vi "UHR-Fleezers Control (host) - 12.7e.vi"() -> ()   [LabVIEW 2012] (continued)
  T23 = typedef "XDNodeRunTimeDep.lvlib/timing_clust.ctl" = cluster{"Expected End [f-1]":u64, "Actual End [f-1]":u64, "Finished Late? [f-1]":bool, "Expected End [i-1]":u64, "Actual End [i-1]":u64, "Finished Late? [i-1]":bool, "Expected Start [i]":u64, "Actual Start [i]":u64, "Expected Start [f]":u64, "Actual Start [f]":u64, "Source Name":string, "Structure Name":string, "Period":i64, "Deadline":i64, "Offset":i64, "Start":i64, "Priority":i32, "Timeout":i32, "Mode":T24, "Wakeup Reason":T25, "Error":errorcluster, "Source Type":string, "Secondary Source Type":string, "Global End Time":u64, "Global Start Time":u64, "Frame Duration":u64, "Iteration Duration":u64, "Assigned CPU":i32, "I/O Scan Engine Mode":u32}
  T24 = typedef "XDNodeRunTimeDep.lvlib/nitl_modes.ctl" = enum32{"No Change", "Process missed periods, maintain original phase", "Discard missed periods, maintain original phase", "Process missed periods, ignore original phase", "Discard missed periods, ignore original phase"}
  T25 = typedef "XDNodeRunTimeDep.lvlib/wakeup.ctl" = enum32{"Normal", "Aborted", "Asynchronous wakeup", "Timing source error", "Timed loop error", "Timeout"}
  T26 = enum16{"big-endian, network order", "native, host order", "little-endian"}
  T27 = enum16{"open", "replace", "create", "open or create", "replace or create", "replace or create with confirmation"}
  T28 = cluster{"Scan Range AOD (nm) 2":dbl, "Step Size AOD (nm) 2":dbl, "Scan Speed AOD (nm/s) 2":dbl, "Number of scans (AOD) 2":u16, "Label":string}
  T29 = cluster{"[0]":dbl, "[1]":dbl, "[2]":dbl, "[3]":dbl, "[4]":dbl, "[5]":dbl}
  T30 = cluster{"Diameter (mm)":dbl, "Units":dbl, "Volume":dbl, "Rate":dbl}
  T31 = enum32{"Status", "Sample Stage", "Syringe Pump", "Trap Control (RF)", "APD Counting", "Fluorescence Laser Control", "Trap AI", "Video", "FPGA"}
  T32 = enum32{"Status", "Sample Stage", "Syringe Pump", "Trap Control (RF)", "APD Counting", "Fluorescence Laser Control", "Trap AI", "Video", "FPGA", "Misc. Configuration"}
  T33 = cluster{"Left":i32, "Top":i32, "Width":u32, "Height":u32}
  T34 = cluster{cluster{"Left":i32, "Top":i32, "Width":u32, "Height":u32}}[]
  T35 = enum32{"setting", "request", "request control", "info", "statistics", "system settings", "I/O sub system", "HRT control", "camera descriptions", "device specific data", "event sub system settings", "event sub system results", "image memory manager"}
  T36 = typedef "AviRefnum.ctl" = refnum<k1>
  T37 = typedef "imagedata.ctl" = cluster{"image type":i32, "image depth":i32, "image":u8[], "mask":u8[], "colors":u32[], "Rectangle":cluster{"left":i16, "top":i16, "right":i16, "bottom":i16}}
  T38 = enum32{"Normal Display", "Dual Display (APD)", "FFT", "High Res Display"}
  T39 = cluster{"Origin Pixel":cluster{"X":sgl, "Y":sgl}, "Angle Relative to Horizontal (deg)":sgl, "Axis Reference":u32}
  T40 = typedef "Simple Grid Descriptor" = cluster{"X Step":sgl, "Y Step":sgl, "Unit":T41}
  T41 = typedef "Image Unit" = enum32{"Undefined", "Angström", "Micrometer", "Millimeter", "Centimeter", "Meter", "Kilometer", "Microinch", "Inch", "Feet", "Nautical miles", "Standard miles", "Steps"}
  T42 = cluster{"averaging mode":u16, "weighting mode":u16, "number of averages":u32}
  T43 = cluster{"dB On (F)":bool, "unwrap phase (F)":bool, "convert to degree (F)":bool}
  T44 = cluster{string, string, string, string, string, string, string, string}
  T45 = cluster{string, string, string, string, string, string, string, string, string, string, string, string}
  T46 = cluster{string, string, string, string, string, string, string, string, string, string, string, string, string}
  T47 = cluster{string, string, string, string, string, string, string, string, string, string, string, string, string, string}
  T48 = cluster{"BD 1 Frequency 1 (MHz)":dbl, "BD 1 Frequency 2 (MHz)":dbl}
  T49 = cluster{"f0":dbl, "df":dbl, "magnitude":dbl[]}[][]
  T50 = cluster{"Comment (data description)":string, "Channel 1 Buffer":string, "Channel 2 Buffer":string, "Channel 3 Buffer":string, "Title":string, "DNA Construct":string, "Bead diameter":dbl, "Name":string}
diagram:
  w18 = u16 10 items=["1.0"=10, "1.5"=15, "2.0"=20] ("stop bits (10: 1 bit)")
  w34 = u16 20 items=["1.0"=10, "1.5"=15, "2.0"=20] ("stop bits (10: 1 bit)")
  w37 = u16 20 items=["1.0"=10, "1.5"=15, "2.0"=20] ("stop bits (10: 1 bit)")
  w45 = u16 20 items=["1.0"=10, "1.5"=15, "2.0"=20] ("stop bits (10: 1 bit)")
  w24 = T19 2 items=["Grayscale (U8)", "Grayscale (I16)", "Grayscale (SGL)", "Complex (CSG)", "RGB (U32)", "HSL (U32)", "RGB (U64)", "Grayscale (U16)"] ("Image Type")
  # "Settings to help prevent AOM/D damage"
  # "Initialize the FPGA DAQ card itself"
  # "Reset the DAQ card."
  # "Specify the DAQ card and the FPGA code to run"
  # "Bottom 1 Harvard"
  # "Top 3 Harvard"
  # "Center Harvard"
  # "Bottom 1 Harvard"
  # "Top 3 Harvard"
  # "Center Harvard"
  n1 = case "Trap X limits" shown="\"AOD3Sets\"" "1axis AOM vs 2 axis AOD" {
    tunnel: [T16 {"Minimum"=0.0, "Maximum"=40.0, "Increment"=0.1} ("Min Max Inc") T16 {"Minimum"=0.0, "Maximum"=40.0, "Increment"=0.1} ("Min Max Inc") T16 {"Minimum"=60.0, "Maximum"=90.0, "Increment"=1.0} ("Min Max Inc")] -> w9
    tunnel: [T16 {"Minimum"=0.0, "Maximum"=45.0, "Increment"=1.0} ("Data Entry Limits") T16 {"Minimum"=0.0, "Maximum"=45.0, "Increment"=1.0} ("Data Entry Limits") T16 {"Minimum"=0.0, "Maximum"=50.0, "Increment"=1.0} ("Data Entry Limits")] -> w7
    frame "2axisAOD" {
      w81 = u16 300 ("DIO count 1 (ticks)")
      # "Amp Limits"
      # "Freq Limits"
      n2 = disable-structure shown="Disabled" {
        frame Disabled {
          w87 = 35.0 ("BD 1 Amplitude 1 (%)")
          w88 = 30.0 ("BD 1 Frequency 1 (MHz)")
          n3 = local write "BD 1 Frequency 1 (MHz)"(w88) -> ()
          n4 = local write "BD 1 Frequency 2 (MHz)"(w88) -> ()
          n5 = local write "BD 1 Amplitude 2 (%)"(w87) -> ()
          n6 = local write "BD 1 Amplitude 1 (%)"(w87) -> ()
          n7 = local write "BD 2 Frequency 1 (MHz)"(w88) -> ()
          n8 = local write "BD 2 Amplitude 1 (%)"(w87) -> ()
          n9 = local write "BD 2 Frequency 2 (MHz)"(w88) -> ()
          n10 = local write "BD 2 Amplitude 2 (%)"(w87) -> ()
        }
        frame Enabled {
        }
      }
      n11 = local write "All FB On/Off"(FALSE ("All FB On/Off")) -> ()
      n12 = local write "BD 2 Delay (Ticks)"(u8 108 ("BD 2 Delay (Ticks)")) -> ()
      n13 = local write "Number Interlace Sets"(u8 2 ("Number Interlace Sets")) -> ()
      n14 = local write "DIO count 2 (ticks)"(w81) -> ()
      n15 = local write "DIO count 1 (ticks)"(w81) -> ()
    }
    frame "AOD3Sets" {
      w89 = u16 200 ("DIO count 1 (ticks)")
      # "Amp Limits"
      # "Freq Limits"
      n16 = disable-structure shown="Disabled" {
        frame Disabled {
          w95 = 35.0 ("BD 1 Amplitude 1 (%)")
          w96 = 30.0 ("BD 1 Frequency 1 (MHz)")
          n17 = local write "BD 1 Frequency 1 (MHz)"(w96) -> ()
          n18 = local write "BD 1 Frequency 2 (MHz)"(w96) -> ()
          n19 = local write "BD 1 Amplitude 2 (%)"(w95) -> ()
          n20 = local write "BD 1 Amplitude 1 (%)"(w95) -> ()
          n21 = local write "BD 2 Frequency 1 (MHz)"(w96) -> ()
          n22 = local write "BD 2 Amplitude 1 (%)"(w95) -> ()
          n23 = local write "BD 2 Frequency 2 (MHz)"(w96) -> ()
          n24 = local write "BD 2 Amplitude 2 (%)"(w95) -> ()
        }
        frame Enabled {
        }
      }
      n25 = local write "All FB On/Off"(FALSE ("All FB On/Off")) -> ()
      n26 = local write "BD 2 Delay (Ticks)"(u8 0 ("BD 2 Delay (Ticks)")) -> ()
      n27 = local write "Number Interlace Sets"(u8 3 ("Number Interlace Sets")) -> ()
      n28 = local write "DIO count 2 (ticks)"(w89) -> ()
      n29 = local write "DIO count 1 (ticks)"(w89) -> ()
    }
    frame "1axis", Default {
      # "Amp Lmits"
      # "Freq Limits"
    }
  }
  n30 = xnode "Open FPGA VI Reference"("resource name"=T18 "750kHzDAQ") -> ("FPGA VI Reference Out"=w14:T20, "error out"=w13:errorcluster)  [unwired: 1 in]
  n31 = xnode "Invoke Method"("FPGA VI Reference In"=w14, "error in"=w13) -> ("FPGA VI Reference Out"=w6:T20, "error out"=→"FPGA error out":errorcluster)
  n32 = flat-sequence "Safety limits on RF frequencies and amplitudes (for AOM protection)" {
    tunnel: [w101] -> w1
    tunnel: [w100] -> w3
    tunnel: [w102] -> w4
    tunnel: [w103] -> w2
    tunnel: w9 -> [w101]
    tunnel: w7 -> [w100]
    tunnel: w6 -> [w99]
    tunnel: [w99] -> w5
    frame #0 {
      w103 = T16 {"Minimum"=0.0, "Maximum"=40.0, "Increment"=0.1} ("Min Max Inc")
      w102 = T16 {"Minimum"=0.0, "Maximum"=45.0, "Increment"=1.0} ("Data Entry Limits")
      n33 = property on="BD 2 Frequency 1 (MHz)" class="DigNum (strict)"("Data Range"=w103) -> ()  [unwired: 2 in, 2 out]
      n34 = property on="BD 2 Frequency 3 (MHz)" class="DigNum (strict)"("Data Range"=w103) -> ()  [unwired: 2 in, 2 out]
      n35 = property on="BD 2 Frequency 2 (MHz)" class="DigNum (strict)"("Data Range"=w103) -> ()  [unwired: 2 in, 2 out]
      n36 = property on="BD 1 Frequency 1 (MHz)" class="DigNum (strict)"("Data Range"=w101) -> ()  [unwired: 2 in, 2 out]
      n37 = property on="BD 1 Frequency 2 (MHz)" class="DigNum (strict)"("Data Range"=w101) -> ()  [unwired: 2 in, 2 out]
      n38 = property on="BD 1 Frequency 3 (MHz)" class="DigNum (strict)"("Data Range"=w101) -> ()  [unwired: 2 in, 2 out]
      n39 = property on="BD 2 Amplitude 1 (%)" class="DigNum (strict)"("Data Range"=w102) -> ()  [unwired: 2 in, 2 out]
      n40 = property on="BD 2 Amplitude 2 (%)" class="DigNum (strict)"("Data Range"=w102) -> ()  [unwired: 2 in, 2 out]
      n41 = property on="BD 2 Amplitude 3 (%)" class="DigNum (strict)"("Data Range"=w102) -> ()  [unwired: 2 in, 2 out]
      n42 = property on="BD 1 Amplitude 3 (%)" class="DigNum (strict)"("Data Range"=w100) -> ()  [unwired: 2 in, 2 out]
      n43 = property on="BD 1 Amplitude 2 (%)" class="DigNum (strict)"("Data Range"=w100) -> ()  [unwired: 2 in, 2 out]
      n44 = property on="BD 1 Amplitude 1 (%)" class="DigNum (strict)"("Data Range"=w100) -> ()  [unwired: 2 in, 2 out]
      "X RF Frequency Limits (MHz)" <- w101
      "X RF Amplitude Limits (%)" <- w100
      "Y RF Amplitude Limits (%)" <- w102
      "Y RF Frequency Limits (MHz)" <- w103
    }
  }
  n45 = stacked-sequence "Host initialization sequence - order matters!" {
    tunnel: w5 -> [_ w106 w204 _ w271 w279 w325 w350 w380]
    tunnel: [_ _ _ _ _ _ _ _ w380] -> w11
    tunnel: [_ _ _ _ _ _ _ _ w379] -> w10
    tunnel: w4 -> [_ _ _ _ _ _ w322 _ _]
    tunnel: w3 -> [_ _ _ _ _ _ w321 _ _]
    tunnel: w2 -> [_ _ _ _ _ _ w320 _ _]
    tunnel: w1 -> [_ _ _ _ _ _ w319 _ _]
    frame #0 {
    }
    frame #1 {
      w139 = 10.0 ("y")
      w140 = 32767.0 ("y")
      w124 = 6.0  # clock mult.
      w123 = 49152000.0  # TCXO frequ.
      # "Initialize some FPGA settings"
      n46 = Build Array("DIO count 1 (ticks)", "DIO count 2 (ticks)", "DIO count 3 (ticks)") -> (w174:u16[])
      n47 = local read "AO1"() -> (w145:dbl)
      n48 = local read "AO2"() -> (w146:dbl)
      n49 = local read "Scan Increment (MHz)"() -> (w128:dbl)
      n50 = property on="AI Count (ticks)" class="DigNum (strict)"("Val(Sgnl)"="AI Count (ticks)") -> ()  [unwired: 2 in, 2 out]
      n51 = local read "Continuous MCL Scanning"() -> (w158:bool)
      n52 = local read "Fast Scan Dir"() -> (w159:bool)
      n53 = local read "Number of scans (MCL)"() -> (w157:u64)
      n54 = Multiply(x=w145, y=w140) -> (x*y=w143:dbl)
      n55 = Multiply(x=w146, y=w140) -> (x*y=w141:dbl)
      n56 = Divide(x=40000000.0, y="AI Count (ticks)") -> (x/y=w163:dbl)
      n57 = Divide(x=w143, y=w139) -> (x/y=w144:dbl)
      n58 = Divide(x=w141, y=w139) -> (x/y=w142:dbl)
      n59 = To Word Integer(number=w144) -> (16bit integer=w147:i16)
      n60 = To Word Integer(number=w142) -> (16bit integer=w148:i16)
      n61 = Not(x=w159) -> (.not. x?=w160:bool)
      n62 = local read "Cycles/step (MCL)"() -> (w156:u64)
      n63 = Multiply(x=w128, y=1000.0) -> (x*y=w121:dbl)
      n64 = local read "Scan steps (MCL)"() -> (w155:u64)
      n65 = local write "Trap Pos FIFO Timeout"(u16 0 ("Trap Pos FIFO Timeout")) -> ()
      n66 = local read "Desired Scan Incr (V)"() -> (w153:dbl)
      n67 = local write "AI rate (Hz)"(w163) -> ()
      n68 = Scale By Power Of 2(n=48, x=w121) -> (x*2^n=w120:dbl)
      n69 = Unbundle By Name(cluster{"output high":i16, "output low":i16} {"output high"=3000, "output low"=0} ("FB output range 1")) -> ("output high"=w193:i16, "output low"=w194:i16)
      n70 = Multiply(x=w123, y=w124) -> (x*y=w125:dbl)
      n71 = Divide(x=w120, y=w125) -> (x/y=w126:dbl)
      n72 = local read "Setpoints (V)"() -> (w113:cluster{"Set 1":dbl, "Set 2":dbl})
      n73 = To Quad Integer(1:w126) -> (0:w129:i64)
      n74 = Multiply(x=w153, y=32767.0) -> (x*y=w151:dbl)
      n75 = Divide(x=w163, y="FPGA Ave.") -> (x/y=w162:dbl)
      n76 = local read "Trap Intensity PID Gains"() -> (w118:T9)
      n77 = local read "Next trap write delay (ticks)"() -> (w197:u8)
      n78 = local read "XY phase ext loop method"() -> (w198:bool)
      n79 = local read "Amp switch delay 2"() -> (w199:u8)
      n80 = local read "BD 2 Delay (Ticks) 2"() -> (w200:u8)
      n81 = local read "BD 1 Delay (ticks) 2"() -> (w201:u8)
      n82 = local write "Ave. Rate (Hz)"(w162) -> ()
      n83 = Reciprocal(x=w162) -> (1/x=w161:dbl)
      n84 = local read "Number Interlace Sets"() -> (w181:u8)
      n85 = Split 1D Array(array=w174, index=w181) -> (first subarray=w172:u16[])  [unwired: 1 out]
      n86 = Add Array Elements(numeric array=w172) -> (sum=w173:u16)
      n87 = local write "Ave. Period (s)"(w161) -> ()
      n88 = local read "# Samples/channel"() -> (w136:u32)
      n89 = local read "Number of F/B Scans (AOD)"() -> (w135:u16)
      n90 = local read "Not-Interlacing Set"() -> (w182:enum32{"Set 1", "Set 2", "Set 3"})
      n91 = To Unsigned Byte Integer(number=w182) -> (unsigned 8bit integer=w176:u8)
      n92 = Index Array(array=w174, index=w176) -> (element=w175:u16)
      n93 = local read "Feedback On/Off"() -> (w110:cluster{"Set 1":bool, "Set 2":bool})
      n94 = local read "BD 2 Delay (Ticks)"() -> (w196:u8)
      n95 = local read "BD 1 Delay (ticks)"() -> (w195:u8)
      n96 = local read "Scan steps (AOD)"() -> (w130:u64)
      n97 = local read "All FB On/Off"() -> (w109:bool)
      n98 = local read "Cycles/step (AOD)"() -> (w131:u64)
      n99 = Divide(x=w151, y=10.0) -> (x/y=w152:dbl)
      n100 = Multiply(x=w130, y=w131) -> (x*y=w132:u64)
      n101 = Unbundle By Name(w118) -> ("proportional gain (Kc)"=w189:i16, "integral gain (Kc*Ts/Ti)"=w190:i16, "derivative gain (Kc*Td/Ts)"=w191:i16)
      n102 = Multiply(x=3276.7, y=w113) -> (x*y=w114:cluster{"Set 1":dbl, "Set 2":dbl})
      n103 = To Word Integer(number=w152) -> (16bit integer=w154:i16)
      n104 = Multiply(x=w132, y=u64 2) -> (x*y=w134:u64)
      n105 = To Word Integer(number=w114) -> (16bit integer=w115:cluster{"Set 1":i16, "Set 2":i16})
      n106 = Multiply(x=w134, y=w135) -> (x*y=w137:u64)
      n107 = local read "Sets to FIFO (Traps)"() -> (w185:T15)
      n108 = Divide(x=w137, y=w136) -> (x/y=w138:dbl)
      n109 = Unbundle By Name(w115) -> ("Set 1"=w116:i16, "Set 2"=w117:i16)
      n110 = local read "2D or 1D Scan"() -> (w171:bool)
      n111 = local write "Data points/scans"(w137) -> ()
      n112 = local read "Scan BD"() -> (w119:bool)
      n113 = And(x=w110, y=w109) -> (x .and. y?=w111:cluster{"Set 1":bool, "Set 2":bool})
      n114 = local write "Data points/scan (f/b)"(w134) -> ()
      n115 = local read "N Acq Sets (Traps + Fl.)"() -> (w167:i16)
      n116 = local write "N sets should be saved"(w138) -> ()
      n117 = local read "FPGA error out"() -> (w105:errorcluster)
      n118 = Unbundle By Name(w111) -> ("Set 1"=w107:bool, "Set 2"=w108:bool)
      n119 = local read "Interlace"() -> (w180:bool)
      n120 = Select(t=w173, s=w180, f=w175) -> (s? t:f=w183:u16)
      n121 = local write "Update Count (MCL)"(w183) -> ()
      n122 = local write "Total Counts (ticks)"(w183) -> ()
      n123 = Unbundle By Name(w185) -> ("Set 1"=w186:bool, "Set 2"=w187:bool, "Set 3"=w188:bool)
      n124 = property on="2D or 1D Scan" class="Bool (strict)"("Val(Sgnl)"=w171) -> ()  [unwired: 2 in, 2 out]
      n125 = xnode "Read/Write Control"("FPGA VI Reference In"=w106, "error in"=w105, "ai count"="AI Count (ticks)", "Interlace ON/OFF"=w180, "Number Interlace Cycles"=w181, "Set 1"=w186, "Set 2"=w187, "Set 3"=w188, "FB On/Off Set 1"=w107, "FB On/Off Set 2"=w108, "Interlace Off Parameters"=w182, "FB Setpoint Set 1"=w116, "FB Setpoint Set 2"=w117, "P1"=w189, "I1"=w190, "D1"=w191, "FB1 output high"=w193, "FB1 output low"=w194, "Cycles per step"=w131, "Scan BD"=w119, "Number of scans"=w135, "Scan steps"=w130, "Scan freq.  increment"=w129, "AO1"=w147, "AO2"=w148, "Scan freq.  increment (MCL)"=w154, "Scan steps (MCL)"=w155, "Cycles per step (MCL)"=w156, "Number of scans (MCL)"=w157, "MCL count"=w183, "Cont. Scan (MCL)"=w158, "MCL Scan Axis"=w160, "1D or 2D Scan?"=w171, "N of AI1 Int Acq Sets"=w167, "Amp switch delay"="Amp switch delay", "Swap F1 and F2"="Swap F1 and F2", "APD to FIFO"=FALSE, "DIO count 1 (ticks)"="DIO count 1 (ticks)", "DIO count 2 (ticks)"="DIO count 2 (ticks)", "DIO count 3 (ticks)"="DIO count 3 (ticks)", "BD 1 Delay (ticks)"=w195, "BD 2 Delay (Ticks)"=w196, "Next trap write delay (ticks)"=w197, "XY phase ext loop method"=w198, "Amp switch delay 2"=w199, "BD 2 Delay (Ticks) 2"=w200, "BD 1 Delay (ticks) 2"=w201) -> ("error out"=w104:errorcluster)  [unwired: 1 in, 1 out]
      n126 = local write "FPGA error out"(w104) -> ()
    }
    frame #2 {
      # "Initialize some more FPGA settings"
      n127 = local read "Laser interlacing mode"() -> (w205:enum32{"Laser ON", "Laser OFF", "Interlace"})
      n128 = local read "Green Laser ON"() -> (w206:bool)
      n129 = local read "Trap Pos. FB Range"() -> (w228:T12)
      n130 = local read "Trap Pos. FB Gains"() -> (w229:T11)
      n131 = Multiply(x="Green Intensity % (FB OFF)", y=655.35) -> (x*y=w211:dbl)
      n132 = local read "Invert laser interlacing"() -> (w248:bool)
      n133 = local read "Trap Pos. AI1 X Pre-scale"() -> (w222:u16)
      n134 = Multiply(x="Green FB Setpoint (mV)", y=3.2767) -> (x*y=w214:dbl)
      n135 = local read "Trap Pos FB Int Count"() -> (w224:u16)
      n136 = local read "Differential FB?"() -> (w227:bool)
      n137 = local read "Neg. TTrig FPGA"() -> (w225:bool)
      n138 = Multiply(x="Red FB Setpoint (mV)", y=3.2767) -> (x*y=w240:dbl)
      n139 = To Unsigned Word Integer(number=w211) -> (unsigned 16bit integer=w213:u16)
      n140 = Multiply(x="Red Intensity % (FB OFF)", y=655.35) -> (x*y=w244:dbl)
      n141 = To Word Integer(number=w214) -> (16bit integer=w216:i16)
      n142 = Unbundle By Name("Green FB Gains") -> ("proportional gain (Kc)"=w237:i16, "integral gain (Kc*Ts/Ti)"=w238:i16, "derivative gain (Kc*Td/Ts)"=w239:i16)
      n143 = Unbundle By Name("Red FB Gains") -> ("proportional gain (Kc)"=w251:i16, "integral gain (Kc*Ts/Ti)"=w252:i16, "derivative gain (Kc*Td/Ts)"=w253:i16)
      n144 = case shown="False" w206 {
        tunnel: w205 -> [_ w256]
        tunnel: [enum32{"Laser ON", "Laser OFF", "Interlace"}."Laser OFF" ("Green laser mode") w256] -> w249
        frame False {
        }
        frame True {
        }
      }
      n145 = To Word Integer(number=w240) -> (16bit integer=w243:i16)
      n146 = Unbundle By Name(w229) -> ("proportional gain (Kc)"=w233:fxp<+/-,16,8>, "integral gain (Kc*Ts/Ti)"=w234:fxp<+/-,16,8>, "derivative gain (Kc*Td/Ts)"=w235:fxp<+/-,16,8>)
      n147 = To Unsigned Word Integer(number=w244) -> (unsigned 16bit integer=w247:u16)
      n148 = Unbundle By Name(w228) -> ("output high"=w230:fxp<+/-,16,1>, "output low"=w232:fxp<+/-,16,1>)
      n149 = local read "Trap Pos FB Monitor\nT1 or T2"() -> (w217:bool)
      n150 = local read "Trap Pos FB Negate Action"() -> (w218:bool)
      n151 = local read "Trap Pos. FB Offset Factor"() -> (w219:i64)
      n152 = local read "Trap Pos. FB Mult Factor"() -> (w220:i64)
      n153 = local read "FPGA error out"() -> (w202:errorcluster)
      n154 = xnode "Read/Write Control"("FPGA VI Reference In"=w204, "error in"=w202, "Invert GI 2"=w248, "Operating Mode 2"=w249, "P3"=w237, "I3"=w238, "D3"=w239, "Green FB Setpoint"=w216, "Green FB On/Off"="Green FB On/Off", "Current Out"=w213, "Green int current ON count adj"="Green int current ON count adj", "Operating Mode"=w249, "Invert GI"=w248, "Trap Pos FB Monitor T1 or T2"=w217, "Trap Pos FB Negate Action"=w218, "Trap Pos. FB Offset Factor"=w219, "Trap Pos. FB Mult Factor"=w220, "Force feedback"=FALSE, "AI1 X Scale"=w222, "Trap Pos to FIFO"=TRUE, "Trap Pos FB Int Count"=w224, "TTrig Negate Pos"=w225, "FB Trig Integrate"="FB Trig Integrate", "Diff FB Measurement?"=w227, "Negate Diff?"="Negate Diff?", "P2"=w233, "I2"=w234, "D2"=w235, "FB2 output high"=w230, "FB2 output low"=w232, "Red FB Setpoint"=w243, "RI Current Out"=w247, "Red Laser Operating Mode"=w249, "RI Operating Mode 2"=w249, "Invert RI 2"=w248, "Invert RI"=w248, "P4"=w251, "I4"=w252, "D4"=w253, "Red FB On/Off"="Red FB On/Off") -> ("error out"=w203:errorcluster)  [unwired: 1 out]
      n155 = local write "FPGA error out"(w203) -> ()
    }
    frame #3 {
      # "Initialize more settings. Should stop using event loops to initialize."
      # "What are these?"
      n156 = stacked-sequence {
        frame #0 {
          w259 = T21."empty" ("mode")
          # "Clear external fluorescence triggering FIFO"
          # "APD loop counts"
          # "Fluorescence loop counts (rates)"
          n157 = local read "APD Integration Time (s)"() -> (w261:dbl)
          n158 = local read "Interlace ON count"() -> (w262:u16)
          n159 = call "Smart Buffer (DBL) 1.vi"("mode"=w259) -> ()  [unwired: 5 in, 6 out]
          n160 = call "Smart Buffer (DBL) 2.vi"("mode"=w259) -> ()  [unwired: 5 in, 6 out]
          n161 = property on="APD Integration Time (s)" class="DigNum (strict)"("Val(Sgnl)"=w261) -> ()  [unwired: 2 in, 2 out]
          n162 = property on="Interlace ON count" class="DigNum (strict)"("Val(Sgnl)"=w262) -> ()  [unwired: 2 in, 2 out]
          "Number of APDs" <- 3.0 ("Number of APDs")
        }
        frame #1 {
          # "Number of APDs affects\nAPD DMA transfer"
          # "General settings for all lasers:"
          # "And includes all laser\nON/OFF settings"
          # "Fluorescent lasers settings:"
          # "Blue laser settings:"
          n163 = local read "Laser interlacing mode"() -> (w264:enum32{"Laser ON", "Laser OFF", "Interlace"})
          n164 = local read "Invert laser interlacing"() -> (w263:bool)
          n165 = local read "Blue FB On/Off"() -> (w265:bool)
          n166 = property on="Blue FB On/Off" class="Bool (strict)"("Val(Sgnl)"=w265) -> ()  [unwired: 2 in, 2 out]
          n167 = property on="Invert laser interlacing" class="Bool (strict)"("Val(Sgnl)"=w263) -> ()  [unwired: 2 in, 2 out]
          n168 = property on="Laser interlacing mode" class="RadioBtnsControl (strict)"("Val(Sgnl)"=w264) -> ()  [unwired: 2 in, 2 out]
        }
        frame #2 {
          w266 = path "C:/Home/wheeler/Comstock-LabView-Link.udl" ("connection information")
          # "Initialize the database connection"
          n169 = call-poly <vilib>:"DB Tools Open Connection.vi"("connection information"=w266) -> ("connection reference"=w267:T17)  [unwired: 7 in, 1 out]
          "connection reference" <- w267
          n170 = local write "connection reference"(w267) -> ()
          n171 = local write "Database link"(w266) -> ()
        }
        frame #3 {
          n172 = Wait (ms)(milliseconds to wait=u32 5000) -> ()  [unwired: 1 out]
        }
      }
      n173 = local write "Offset (nm)"(0.0 ("Offset (nm)")) -> ()
      n174 = local write "Bead Mean (nm)"(0.0 ("Bead Mean (nm)")) -> ()
    }
    frame #4 {
      # "Set FIFO size and run FPGA"
      n175 = local read "FPGA error out"() -> (w270:errorcluster)
      n176 = xnode "Invoke Method"("FPGA VI Reference In"=w271, "error in"=w270, "Requested Depth"="Trap AI FIFO Depth") -> ("FPGA VI Reference Out"=w275:T20, "error out"=w276:errorcluster)  [unwired: 1 out]
      n177 = xnode "Invoke Method"("FPGA VI Reference In"=w275, "error in"=w276, "Requested Depth"="Trap Position FIFO Depth") -> ("FPGA VI Reference Out"=w273:T20, "error out"=w272:errorcluster)  [unwired: 1 out]
      n178 = xnode "Invoke Method"("FPGA VI Reference In"=w273, "error in"=w272) -> ("error out"=w269:errorcluster)  [unwired: 1 in, 1 out]
      n179 = local write "FPGA error out"(w269) -> ()
    }
    frame #5 {
      # "Adjust FPGA timing loop phases"
      n180 = flat-sequence "Initial FPGA Loop Relative Phase Adjustment" {
        tunnel: "Initial Phase Adjustment (AI1)" -> [w310]
        tunnel: "Initial Phase Adjustment (GI)" -> [w309]
        tunnel: "Initial Phase Adj. (MCL)" -> [w308]
        tunnel: [w311] -> w295
        tunnel: [w307] -> w294
        tunnel: "Initial Phase Adjustment (APD Acq)" -> [w306]
        tunnel: "Initial Phase Adjustment (APD 1 Gate)" -> [w305]
        tunnel: "Initial Phase Adjustment (Green FB)" -> [w304]
        tunnel: "Initial Phase Adjustment (GI) 2" -> [w303]
        tunnel: "Initial Phase Adjustment (APD 2 Gate)" -> [w302]
        tunnel: "Initial Phase Adjustment (RI)" -> [w301]
        tunnel: "Initial Phase Adjustment (BI DO)" -> [w300]
        tunnel: "Initial Phase Adjustment (BI AO)" -> [w299]
        tunnel: "Initial Phase Adjustment (APD 3 Gate)" -> [w298]
        tunnel: w279 -> [w297]
        tunnel: w295 -> [w313]
        tunnel: [w314] -> w293
        tunnel: w294 -> [w314]
        tunnel: [w313] -> w292
        tunnel: w293 -> [w318]
        tunnel: w292 -> [w317]
        tunnel: [w315] -> w278
        frame #0 {
          n181 = local read "FPGA error out"() -> (w296:errorcluster)
          n182 = xnode "Read/Write Control"("FPGA VI Reference In"=w297, "error in"=w296, "Phase count adjustment"=w310, "Phase count adjustment (GI)"=w309, "Phase count adjustment (MCL)"=w308, "Phase Count Adjustment (APD Acq)"=w306, "Phase count adjustment (APD 1 Gate)"=w305, "Phase count adjustment (APD 2 Gate)"=w302, "Phase count adjustment (Green FB)"=w304, "Phase count adjustment (GI) 2"=w303, "Phase count adjustment (RI)"=w301, "Phase count adjustment (BI AO)"=w299, "Phase count adjustment (BI D)"=w300, "Phase count adjustment (APD 3 Gate)"=w298) -> ("FPGA VI Reference Out"=w307:T20, "error out"=w311:errorcluster)
        }
        frame #1 {
          n183 = Wait (ms)(milliseconds to wait=u32 100) -> ()  [unwired: 1 out]
        }
        frame #2 {
          w316 = TRUE
          n184 = xnode "Read/Write Control"("FPGA VI Reference In"=w318, "error in"=w317, "+ phase"=w316, "+ phase (GI)"=w316, "+ phase (MCL)"=w316, "+ phase (APD Acq)"=w316, "+ phase (APD 1 Gate)"=w316, "+ phase (APD 2 Gate)"=w316, "+ phase (Green FB)"=w316, "+ phase (GI) 2"=w316, "+ phase (RI)"=w316, "+ phase (BI AO)"=w316, "+ phase (BI D)"=w316, "+ phase (APD 3 Gate)"=w316) -> ("error out"=w315:errorcluster)  [unwired: 1 out]
        }
      }
      n185 = local write "FPGA error out"(w278) -> ()
    }
    frame #6 {
      # "Initialize trap RF synth board and set initial frequencies and amplitudes"
      n186 = local read "FPGA error out"() -> (w324:errorcluster)
      n187 = call "Initialize RF boards - interlace 3.vi"("error in"=w324, "FPGA VI Reference In"=w325) -> ("error out"=w326:errorcluster, "FPGA VI Reference Out"=w347:T20)
      n188 = call "set RF board frequency - interlace.vi"("Board 2 Frequency Limits"=w320, "Board 1 Frequency Limits"=w319, "error in"=w326, "FPGA VI Reference In"=w347, "Board 2 Frequency 3 (MHz)"="BD 2 Frequency 3 (MHz)", "Board 1 Frequency 3 (MHz)"="BD 1 Frequency 3 (MHz)", "Board 2 Frequency 2 (MHz)"="BD 2 Frequency 2 (MHz)", "Board 2 Frequency 1 (MHz)"="BD 2 Frequency 1 (MHz)", "Board 1 Frequency 2 (MHz)"="BD 1 Frequency 2 (MHz)", "Board 1 Frequency 1  (MHz)"="BD 1 Frequency 1 (MHz)") -> ("error out"=w330:errorcluster, "FPGA VI Reference Out"=w329:T20)
      n189 = call "set RF board amplitude - interlace.vi"("Board 2 Amplitude Limits"=w322, "Board 1 Amplitude Limits"=w321, "error in"=w330, "FPGA VI Reference In"=w329, "Board 2 Amplitude 3 (%)"="BD 2 Amplitude 3 (%)", "Board 1 Amplitude 3 (%)"="BD 1 Amplitude 3 (%)", "Board 2 Amplitude 2 (%)"="BD 2 Amplitude 2 (%)", "Board 2 Amplitude 1 (%)"="BD 2 Amplitude 1 (%)", "Board 1 Amplitude 2 (%)"="BD 1 Amplitude 2 (%)", "Board 1 Amplitude 1 (%)"="BD 1 Amplitude 1 (%)") -> ("error out"=w323:errorcluster)  [unwired: 1 out]
      n190 = Subtract(x="BD 1 Frequency 1 (MHz)", y="BD 1 Frequency 2 (MHz)") -> (x-y=w337:dbl)
      n191 = Subtract(x="BD 2 Frequency 1 (MHz)", y="BD 2 Frequency 2 (MHz)") -> (x-y=w338:dbl)
      n192 = local write "FPGA error out"(w323) -> ()
      n193 = Square(x=w338) -> (x^2=w340:dbl)
      n194 = Square(x=w337) -> (x^2=w339:dbl)
      n195 = Add(x=w339, y=w340) -> (x+y=w341:dbl)
      n196 = Square Root(x=w341) -> (sqrt(x)=w342:dbl)
      n197 = local write "Trap Delta (MHz)"(w342) -> ()
    }
    frame #7 {
      n198 = local read "FPGA error out"() -> (w349:errorcluster)
      n199 = flat-sequence {
        tunnel: [w364] -> w354
        tunnel: [w363] -> w353
        tunnel: w350 -> [w356]
        tunnel: w349 -> [w355]
        tunnel: [w368] -> w352
        tunnel: w354 -> [w368]
        tunnel: [w367] -> w351
        tunnel: w353 -> [w367]
        tunnel: w352 -> [w376]
        tunnel: w351 -> [w375]
        tunnel: [w370] -> w348
        frame #0 {
          w357 = FALSE ("Retract Pump 3")
          n200 = local read "Trap 1 (ON/OFF)"() -> (w358:bool)
          n201 = xnode "Read/Write Control"("FPGA VI Reference In"=w356, "error in"=w355, "Direct RF Box  Communication"=FALSE) -> ("FPGA VI Reference Out"=w364:T20, "error out"=w363:errorcluster)
          n202 = local write "Saving..."(FALSE ("Saving Data")) -> ()
          n203 = local write "Stop All"(FALSE ("Stop All")) -> ()
          n204 = local write "Retract Pump 1"(w357) -> ()
          n205 = local write "Retract Pump 3"(w357) -> ()
          n206 = local write "Index"(1.0 ("Index")) -> ()
          n207 = property on="Trap 1 ON" class="Bool (strict)"("Value"=w358) -> ()  [unwired: 2 in, 2 out]
          "Manipulating Trap" <- FALSE ("Manipulating Trap")
        }
        frame #1 {
          n208 = local read "Trap 2 (ON/OFF)"() -> (w366:bool)
          n209 = Wait (ms)(milliseconds to wait=u32 10) -> ()  [unwired: 1 out]
          n210 = property on="Trap 2 ON" class="Bool (strict)"("Val(Sgnl)"=w366) -> ()  [unwired: 2 in, 2 out]
        }
        frame #2 {
          n211 = local read "Scan Range (nm)"() -> (w371:dbl)
          n212 = xnode "Read/Write Control"("FPGA VI Reference In"=w376, "error in"=w375, "FPGA Controls  RF Box"=TRUE ("Direct RF Box  Communication")) -> ("error out"=w370:errorcluster)  [unwired: 1 out]
          n213 = call "Update messages.vi"("Message to add"="UHR-Fleezers ready.", "Old message string"="") -> ("New message string"=w374:string)
          n214 = local write "Messages"(w374) -> ()
          n215 = property on="Scan Range (nm)" class="DigNum (strict)"("Val(Sgnl)"=w371) -> ()  [unwired: 2 in, 2 out]
        }
      }
      n216 = local write "FPGA error out"(w348) -> ()
    }
    frame #8 {
      # "Wait 5 s for all the event loops still being executed to finish."
      n217 = Wait (ms)(milliseconds to wait=u32 5000) -> ()  [unwired: 1 out]
      n218 = local read "FPGA error out"() -> (w379:errorcluster)
    }
  }
  n219 = call-poly "VISA Configure Serial Port"("VISA resource name"="VISA resource name", "baud rate (9600)"=u32 115200, "stop bits (10: 1 bit)"=w18) -> ("VISA resource name out"=w17:refnum<visa-resource-name>, "error out"=w16:errorcluster)  [unwired: 4 in, 7 out]
  n220 = call-poly "VISA Configure Serial Port"("VISA resource name"="Bottom  1 Harvard Syringe Pump Serial Port", "baud rate (9600)"=u32 115200, "stop bits (10: 1 bit)"=w34) -> ("VISA resource name out"=w30:refnum<visa-resource-name>, "error out"=w29:errorcluster)  [unwired: 4 in, 7 out]
  n221 = call-poly "VISA Configure Serial Port"("VISA resource name"="Top 3 Harvard Syringe Pump Serial Port", "baud rate (9600)"=u32 115200, "stop bits (10: 1 bit)"=w37) -> ("VISA resource name out"=w32:refnum<visa-resource-name>, "error out"=w31:errorcluster)  [unwired: 4 in, 7 out]
  n222 = call-poly "VISA Configure Serial Port"("VISA resource name"="Sample Chamber Stage Serial Port") -> ("VISA resource name out"=w58:refnum<visa-resource-name>, "error out"=w59:errorcluster)  [unwired: 5 in, 8 out]
  "Stage Control Serial Error" <- w59
  n223 = local write "Blue Error Out"(w16) -> ()
  n224 = call-poly "VISA Configure Serial Port"("VISA resource name"="Center Harvard Syringe Pump Serial Port", "baud rate (9600)"=u32 115200, "stop bits (10: 1 bit)"=w45) -> ("VISA resource name out"=w42:refnum<visa-resource-name>, "error out"=w43:errorcluster)  [unwired: 4 in, 7 out]
  n225 = call "IMAQ Create"("Image Name"="APD 1 Image", "Image Type"=w24) -> ("New Image"=w51:T2)  [unwired: 3 in, 1 out]
  n226 = call "IMAQ Create"("Image Name"="APD 2 Image", "Image Type"=w24) -> ("New Image"=w50:T2)  [unwired: 3 in, 1 out]
  n227 = call "IMAQ Create"("Image Name"="APD 3 Image", "Image Type"=w24) -> ("New Image"=w23:T2)  [unwired: 3 in, 1 out]
  n228 = call "IMAQ Create"("Image Name"="Det. X Image", "Image Type"=w24) -> ("New Image"=w49:T2)  [unwired: 3 in, 1 out]
  n229 = call "IMAQ Create"("Image Name"="Det. Y Image", "Image Type"=w24) -> ("New Image"=w48:T2)  [unwired: 3 in, 1 out]
  n230 = Bundle("New Image"=w51, "New Image"=w50, "New Image"=w23, "New Image"=w49, "New Image"=w48) -> (w47:T22)  [unwired: 1 in]
  n231 = node-c288(2 ("Processor")) -> (w66:T23)  [unwired: 3 out]
  n232 = node-c288() -> (w22:T23)  [unwired: 4 out]
  n233 = node-c288() -> (w54:T23)  [unwired: 4 in]
  n234 = node-c288(3 ("Processor")) -> (w64:T23)  [unwired: 3 out]
  n235 = node-c288() -> (w68:T23)  [unwired: 4 out]
  n236 = while "Duncan's play event loop" {
    stop <- w382 stop-if-true
    n237 = Create User Event(user event datatype=TRUE ("Boolean")) -> (user event=w383:refnum<user-event>)  [unwired: 1 in, 1 out]
    n238 = Create User Event(user event datatype=TRUE ("Boolean")) -> (user event=w390:refnum<user-event>)  [unwired: 1 in, 1 out]
    n239 = global write "Global for fluorescence simulation mean (30 samples), (power series).vi" "Red Signal"(w383) -> ()
    n240 = global write "Global for fluorescence simulation mean (30 samples), (power series).vi" "Green Signal"(w390) -> ()
    n241 = register-events(w390, w383) -> (reference out=w389:refnum<event-registration>)  [unwired: 2 in, 1 out]
    n242 = event shown="[1] \"Get Fluorophore\": Value Change" {
      selector: w389 -> [_ _ _ _]
      dyn-events: _ -> [_ _ _ _]
      timeout: 100 -> [_ _ _ _]
      event Timeout {
        n243 = event-data() -> ()  [unwired: 1 in, 2 out]
      }
      event "Get Fluorophore": Value Change {
        n244 = event-data() -> ("OldVal"=w392:bool)  [unwired: 1 in, 4 out]
        n245 = case shown="True" w392 {
          selector: w392 -> [_ w393]
          frame False {
          }
          frame True {
            n246 = property on="Move to Position 3" class="Bool"("Val(Sgnl)"=w393) -> ()  [unwired: 2 in, 2 out]
            n247 = case shown="1" "Numeric" {
              frame 0, Default {
              }
              frame 1 {
                n248 = property on="Green Laser ON" class="Bool (strict)"("Val(Sgnl)"=TRUE ("Value (Signaling)")) -> ()  [unwired: 2 in, 2 out]
              }
              frame 2 {
                n249 = property on="Red Laser ON" class="Bool (strict)"("Val(Sgnl)"=TRUE) -> ()  [unwired: 2 in, 2 out]
              }
            }
          }
        }
      }
      event User Event {
        n250 = event-data() -> ("Boolean"=w397:bool)  [unwired: 1 in, 3 out]
        "Green Fluorophore" <- w397
        n251 = property on="Get Fluorophore" class="Bool (strict)"("Val(Sgnl)"=w397) -> ()  [unwired: 2 in, 2 out]
      }
      event User Event {
        n252 = event-data() -> ("Boolean"=w398:bool)  [unwired: 1 in, 3 out]
        "Red Fluorophore" <- w398
        n253 = property on="Get Fluorophore" class="Bool (strict)"("Val(Sgnl)"=w398) -> ()  [unwired: 2 in, 2 out]
      }
    }
    n254 = property on="Get Fluorophore" class="Bool (strict)"("Val(Sgnl)"="Get Fluorophore") -> ()  [unwired: 2 in, 2 out]
    n255 = Wait (ms)(milliseconds to wait=u32 100) -> ()  [unwired: 1 out]
    n256 = local read "Stop All"() -> (w381:bool)
    n257 = Or(x=w381, y="stop") -> (x .or. y?=w382:bool)
  }
  n258 = timed-loop "Basic control parameters (all FPGA settings, other basic controls)" {
    shift-right: [w406] -> _
    shift-left: errorcluster {"status"=FALSE, "code"=0, "source"=""} ("error out") -> [_]
    tunnel: [w405] -> _
    timing: w66 -> [_]
    timing-out: [_] -> w65
    tunnel: w42 -> [w404]
    tunnel: w32 -> [w403]
    tunnel: w31 -> [w402]
    tunnel: w30 -> [w401]
    tunnel: w29 -> [w400]
    tunnel: w5 -> [w399]
    stop <- w405 stop-if-true
    n259 = node-c288() -> ()  [unwired: 2 out]
    n260 = event shown="[2] \"Detector Type\": Value Change" {
      selector: _ -> [_ _ _ _ _ _ _ _ _ _ _ _ _ _ _ _ _ _ _ _ _ _ _ _ _ _ _ _ _ _ _ _ _ _ _ _ _ _ _ _ _ _ _ _ _ _ _ _ _ _ _ _ _ _ _ _ _ _ _ _ _ _ _ _ _ _ _ _ _ _ _ _ _ _]
      dyn-events: _ -> [_ _ _ _ _ _ _ _ _ _ _ _ _ _ _ _ _ _ _ _ _ _ _ _ _ _ _ _ _ _ _ _ _ _ _ _ _ _ _ _ _ _ _ _ _ _ _ _ _ _ _ _ _ _ _ _ _ _ _ _ _ _ _ _ _ _ _ _ _ _ _ _ _ _]
      timeout: _ -> [_ _ _ _ _ _ _ _ _ _ _ _ _ _ _ _ _ _ _ _ _ _ _ _ _ _ _ _ _ _ _ _ _ _ _ _ _ _ _ _ _ _ _ _ _ _ _ _ _ _ _ _ _ _ _ _ _ _ _ _ _ _ _ _ _ _ _ _ _ _ _ _ _ _]
      tunnel: [w446 _ _ _ w476 _ _ _ _ _ _ w547 _ _ w615 w617 w626 w628 w698 _ w717 w741 w761 w781 w800 w824 w853 _ w858 w952 w956 w993 _ w1027 w1030 w1033 w1043 w1046 _ w1053 _ _ _ _ _ _ _ _ _ _ _ _ _ _ _ _ _ w1430 _ _ _ _ w1466 _ _ _ _ _ _ _ _ _ _ _] -> w406
      tunnel: [_ _ _ _ _ _ _ _ _ w532 _ _ _ _ _ _ _ _ _ _ _ _ _ _ _ _ _ _ _ _ _ _ _ _ _ _ _ _ _ _ _ _ _ _ _ _ _ _ _ _ _ _ _ _ _ _ _ _ _ _ _ _ _ _ _ _ _ _ _ _ _ _ _ _] -> w405
      tunnel: [_ _ _ _ _ _ _ "Round T1 X" _ _ _ _ _ _ _ _ _ _ _ _ _ _ _ _ _ _ _ _ _ _ _ _ _ _ _ _ _ _ _ _ _ _ _ _ _ _ _ _ _ _ _ _ _ _ _ _ _ _ _ _ _ _ _ _ _ _ _ _ _ _ _ _ _ _] -> _
      tunnel: [_ _ _ "Adjust Scale\nto Mean" _ _ _ _ _ _ _ _ _ _ _ _ _ _ _ _ _ _ _ _ _ _ _ _ "Test ttrig" _ _ _ _ _ _ _ _ _ _ _ _ _ _ _ _ _ _ "Flush Sample" "Flush Pump 3" "Flush Pump 1" "Clear Volume" _ _ _ _ _ _ _ _ _ _ _ _ _ _ _ _ _ _ _ _ _ _ _] -> _
      tunnel: [_ _ _ _ _ _ _ _ "Round T2 X" _ "Delayed Interlace Start" _ _ _ _ _ _ _ _ _ _ _ _ _ _ _ _ _ _ _ _ _ _ _ _ _ _ _ _ _ _ _ _ _ _ _ _ _ _ _ _ _ _ _ _ _ _ _ _ _ _ _ _ _ _ _ _ _ _ _ _ _ _ _] -> _
      tunnel: w404 -> [_ _ _ _ _ _ _ _ _ _ _ _ _ _ _ _ _ _ _ _ _ _ _ _ _ _ _ _ _ _ _ _ _ _ _ _ _ _ _ _ _ _ _ w1210 w1217 w1224 w1229 w1238 _ _ w1344 _ _ _ _ _ _ _ _ _ _ _ _ _ _ _ _ _ _ _ _ _ _ _]
      tunnel: w403 -> [_ _ _ _ _ _ _ _ _ _ _ _ _ _ _ _ _ _ _ _ _ _ _ _ _ _ _ _ _ _ _ _ _ _ _ _ _ _ _ _ _ w1127 _ _ _ _ _ _ w1282 _ _ w1350 _ w1359 _ w1373 _ _ _ _ _ _ _ _ _ _ _ _ _ _ _ _ _ _]
      tunnel: w402 -> [_ _ _ _ _ _ _ _ _ _ _ _ _ _ _ _ _ _ _ _ _ _ _ _ _ _ _ _ _ _ _ _ _ _ _ _ _ _ _ _ _ _ _ _ _ _ _ _ _ _ _ _ _ _ _ _ _ _ _ _ _ _ _ _ _ _ _ _ _ _ _ _ _ _]
      tunnel: w401 -> [_ _ _ _ _ _ _ _ _ _ _ _ _ _ _ _ _ _ _ _ _ _ _ _ _ _ _ _ _ _ _ _ _ _ _ _ _ _ _ _ w1064 _ _ _ _ _ _ _ _ w1312 _ _ w1355 _ w1366 _ w1398 _ _ _ _ _ _ _ _ _ _ _ _ _ _ _ _ _]
      tunnel: w400 -> [_ _ _ _ _ _ _ _ _ _ _ _ _ _ _ _ _ _ _ _ _ _ _ _ _ _ _ _ _ _ _ _ _ _ _ _ _ _ _ _ _ _ _ _ _ _ _ _ _ _ _ _ _ _ _ _ _ _ _ _ _ _ _ _ _ _ _ _ _ _ _ _ _ _]
      tunnel: w399 -> [w409 _ _ _ w475 _ w501 _ _ _ _ w538 _ _ w593 w616 w621 w627 w663 _ w706 w739 w742 w762 w782 w801 w829 w854 w856 w860 w953 w957 _ w1024 w1028 w1031 w1041 w1044 _ w1052 _ _ _ _ _ _ _ _ _ _ _ _ _ _ _ _ _ w1423 _ w1444 _ w1450 w1465 _ w1472 w1474 w1481 w1495 w1510 _ w1519 _ w1539 _]
      event "AI Count (ticks)", "Sets to FIFO (Traps)", "Save ave N", "FPGA Ave.", "# Samples/channel", "N sets to save": Value Change {
        # "So that if 'Save ave N' is updated, the AOD scanning code updates too."
        n261 = event-data() -> ()  [unwired: 6 out]
        n262 = local read "AI Count (ticks)"() -> (w430:u16)
        n263 = Unbundle By Name("Sets to FIFO (Traps)") -> ("Set 1"=w413:bool, "Set 2"=w412:bool, "Set 3"=w411:bool)
        n264 = Boolean To (0,1)(Boolean="Sets to FIFO (Traps)") -> (0, 1=w438:cluster{"Set 1":i16, "Set 2":i16, "Set 3":i16})
        n265 = xnode "Read/Write Control"("FPGA VI Reference In"=w409, "ai count"=w430, "Set 1"=w413, "Set 2"=w412, "Set 3"=w411, "N of AI1 Int Acq Sets"="N Acq Sets (Traps + Fl.)") -> ("error out"=w446:errorcluster)  [unwired: 1 in, 1 out]
        n266 = Cluster To Array(cluster=w438) -> (array=w437:i16[])
        n267 = To Unsigned Long Integer(number=w437) -> (unsigned 32bit integer=w419:u32[])
        n268 = local read "Scan steps (AOD)"() -> (w439:u64)
        n269 = Multiply(x=w430, y="N Acq Sets (Traps + Fl.)") -> (x*y=w428:u16)
        n270 = Divide(x=40000000.0, y=w430) -> (x/y=w422:dbl)
        "AI rate (Hz)" <- w422
        "Ave. Rate (Hz)" <- w422
        n271 = Add Array Elements(numeric array=w419) -> (sum=w431:u32)
        "Trap Sets" <- w431
        n272 = Reciprocal(x=w422) -> (1/x=→"Ave. Period (s)":dbl)
        n273 = property on="Scan steps (AOD)" class="DigNum (strict)"("Val(Sgnl)"=w439) -> ()  [unwired: 2 in, 2 out]
        n274 = Divide(x=w422, y="N Acq Sets (Traps + Fl.)") -> (x/y=w443:dbl)
        "Data Rate (Hz)" <- w443
        n275 = Reciprocal(x=w443) -> (1/x=→"Data Period (s)":dbl)
        n276 = local read "Save ave N"() -> (w442:dbl)
        n277 = Divide(x=w443, y=w442) -> (x/y=w441:dbl)
        "Save Data Rate (Hz)" <- w441
        n278 = Reciprocal(x=w441) -> (1/x=→"Save Data Period (s)":dbl)
        n279 = Multiply(x=w428, y="# Samples/trap") -> (x*y=w426:u32)
        "Counts/DMA" <- w426
        n280 = property on="Trap Disp. Downsample" class="DigNum (strict)"("Maximum"="# Samples/trap") -> ()  [unwired: 2 in, 2 out]
        n281 = Multiply(x=w431, y="# Samples/trap") -> (x*y=w420:u32)
        "# Samples/channel" <- w420
        n282 = Multiply(x=w420, y=u32 8) -> (x*y=→"Trap AI Elements/DMA read":u32)
        n283 = local read "APD Int. Count"() -> (w427:u32)
        n284 = Multiply(x=w420, y=u32 3) -> (x*y=→"Trap Pos Elements/DMA read":u32)
        n285 = Divide(x=w426, y=w427) -> (x/y=w417:dbl)
        "APD Samples/FIFO Acq." <- w417
        n286 = Divide(x=w426, y=40000000.0) -> (x/y=w424:dbl)
        "DMA Update Period (s)" <- w424
        n287 = local read "Number of APDs"() -> (w410:u8)
        n288 = Multiply(x=w410, y=w417) -> (x*y=→"APD Elements/DMA read":dbl)
        n289 = property on="APD Disp. Downsample" class="DigNum (strict)"("Maximum"=w417) -> ()  [unwired: 2 in, 2 out]
        n290 = local read "N sets to save"() -> (w436:u32)
        n291 = Multiply(x=w424, y=w436) -> (x*y=→"Total Time (s)":dbl)
        "FPGA Averaging" <- FALSE ("FPGA Averaging")
      }
      event "Remove Offset": Value Change {
        n292 = event-data() -> ()  [unwired: 7 out]
        n293 = local write "Remove Offset"(FALSE ("Remove Offset")) -> ()
        n294 = local read "Bead Mean (nm)"() -> (w448:dbl)
        n295 = local read "Offset (nm)"() -> (w449:dbl)
        n296 = Add(x=w448, y=w449) -> (x+y=w447:dbl)
        n297 = local write "Offset (nm)"(w447) -> ()
        n298 = disable-structure shown="Disabled" {
          frame Disabled {
            n299 = local read "Bead Mean (nm)"() -> (w454:dbl)
            n300 = Add(y=w454) -> (x=w453:dbl, x+y=w452:dbl)
            n301 = Subtract(x=w454, y=w453) -> (x-y=w451:dbl)
            n302 = property on="Bead Separation" class="WFChart (strict)"("YScale.Minimum"=w451) -> ()  [unwired: 2 in, 2 out]
            n303 = property on="Bead Separation" class="WFChart (strict)"("YScale.Maximum"=w452) -> ()  [unwired: 2 in, 2 out]
          }
          frame Enabled {
          }
        }
      }
      event "Detector Type": Value Change {
        n304 = event-data() -> ()  [unwired: 7 out]
        n305 = local read "AI labels"() -> (w456:string[])
        n306 = property on="High Res. Display" class="Ring (strict)"("Strings []"=w456) -> ()  [unwired: 2 in, 2 out]
        n307 = Build Array (concatenate)(w456, "none") -> (w457:string[])
        n308 = property on="FFT 1 Choice 1" class="Ring (strict)"("Strings []"=w457) -> ()  [unwired: 2 in, 2 out]
        n309 = property on="FFT 1 Choice 2" class="Ring (strict)"("Strings []"=w457) -> ()  [unwired: 2 in, 2 out]
        n310 = property on="FFT 2 Choice 1" class="Ring (strict)"("Strings []"=w457) -> ()  [unwired: 2 in, 2 out]
        n311 = property on="FFT 2 Choice 2" class="Ring (strict)"("Strings []"=w457) -> ()  [unwired: 2 in, 2 out]
        n312 = Bundle("APD 1", "APD 2", "APD 3") -> (w460:cluster{string, string, string})  [unwired: 1 out]
        n313 = Cluster To Array(cluster=w460) -> (array=w458:string[])
        n314 = Build Array (concatenate)(w458, w457) -> (w462:string[])
        n315 = Array Size(array=w462) -> (size(s)=w463:i32)
        n316 = property on="Signals to Plot" class="LstBox (strict)"("Item Names"=w462) -> ()  [unwired: 2 in, 2 out]
        n317 = property on="Signals to Plot" class="LstBox (strict)"("Number of Rows"=w463) -> ()  [unwired: 2 in, 2 out]
        n318 = property on="All Signals" class="WFChart (strict)"("LegNumRows"=w463) -> ()  [unwired: 2 in, 2 out]
      }
      event "Adjust Scale\nto Mean": Value Change {
        n319 = event-data() -> ()  [unwired: 7 out]
        n320 = local read "APD 1 Rate (Hz)"() -> (w472:dbl)
        n321 = Multiply(x=1000.0, y="Above (kHz)") -> (x*y=w470:dbl)
        n322 = Multiply(x=1000.0, y="Below (kHz)") -> (x*y=w468:dbl)
        n323 = Add(x=w470, y=w472) -> (x+y=w465:dbl)
        n324 = Subtract(x=w472, y=w468) -> (x-y=w466:dbl)
        n325 = property on="APD Chart" class="WFChart (strict)"("YScale.Minimum"=w466) -> ()  [unwired: 2 in, 2 out]
        n326 = property on="APD Chart" class="WFChart (strict)"("YScale.Maximum"=w465) -> ()  [unwired: 2 in, 2 out]
      }
      event "Phase adj. (AI1)", "+ phase (AI1)", "- phase (AI1)": Value Change {
        n327 = event-data() -> ()  [unwired: 7 out]
        n328 = Negate(x="Phase adj. (AI1)") -> (-x=w483:i16)
        n329 = Select(t=w483, s="- phase (AI1)", f="Phase adj. (AI1)") -> (s? t:f=w482:i16)
        n330 = xnode "Read/Write Control"("FPGA VI Reference In"=w475, "Phase count adjustment"=w482) -> ("FPGA VI Reference Out"=w481:T20, "error out"=w480:errorcluster)  [unwired: 2 in]
        n331 = Or(x="- phase (AI1)", y="+ phase (AI1)") -> (x .or. y?=w477:bool)
        n332 = xnode "Read/Write Control"("FPGA VI Reference In"=w481, "error in"=w480, "+ phase"=w477) -> ("error out"=w476:errorcluster)  [unwired: 1 in, 1 out]
      }
      event "Signals to Plot": Double Click {
        w487 = u32 9868950 ("Color Box")
        n333 = event-data() -> ("Row"=w489:i32)  [unwired: 9 out]
        n334 = property on="All Signals" class="WFChart (strict)"("Active Plot"=w489) -> (error out=w500:errorcluster)  [unwired: 2 in, 1 out]
        n335 = property on="All Signals" class="WFChart (strict)" props=["Plot", "Visible?", "Plot", "Plot Color"](error in=w500) -> (error out=w499:errorcluster, "Plot.Visible?"=w498:bool)  [unwired: 1 in, 2 out]
        n336 = Select(t=FALSE ("Plot.Visible"), s=w498, f=TRUE ("Plot.Visible")) -> (s? t:f=w493:bool)
        n337 = property on="All Signals" class="WFChart (strict)"(error in=w499, "Plot.Visible?"=w493) -> (error out=w495:errorcluster)  [unwired: 1 in, 1 out]
        n338 = property on="All Signals" class="WFChart (strict)"(error in=w495) -> (error out=w490:errorcluster, "Plot.Plot Color"=w494:u32)  [unwired: 1 in, 1 out]
        n339 = property on="Signals to Plot" class="LstBox (strict)"(error in=w490, "Active Row"=w489) -> (error out=w488:errorcluster)  [unwired: 1 in, 1 out]
        n340 = Select(t=w494, s=w493, f=u32 0) -> (s? t:f=w491:u32)
        n341 = property on="Signals to Plot" class="LstBox (strict)"(error in=w488, "CellFontColor"=w491, "SelColor"=w487, "CellBG"=w487, "CellFontSize"=u32 20 ("Active Row:Cell Font:Size"), "CellFontBold"=TRUE ("Active Row:Cell Font:Bold")) -> ()  [unwired: 1 in, 2 out]
      }
      event "BD 1 Frequency 1 (MHz)", "BD 1 Frequency 2 (MHz)", "BD 1 Frequency 3 (MHz)", "BD 2 Frequency 1 (MHz)", "BD 2 Frequency 2 (MHz)", "BD 2 Frequency 3 (MHz)", "Trap Delta (MHz)", "Update all trap values": Value Change {
        # "This is so you can set trap frequencies\nvia local variables and then update\nall at once"
        n342 = event-data() -> ("CtlRef"=w505:refnum<vi>)  [unwired: 6 out]
        n343 = control-ref of="Trap Delta (MHz)"() -> (w504:refnum<vi>)
        n344 = Equal?(x=w504, y=w505) -> (x = y?=w503:bool)
        n345 = local write "Update all trap values"(FALSE ("Update all trap values")) -> ()
        n346 = case shown="False" "Oscillate Set 1" {
          tunnel: w503 -> [w509 _]
          tunnel: w501 -> [w507 _]
          frame False {
            n347 = local read "BD 1 Frequency 2 (MHz)"() -> (w513:dbl)
            n348 = local read "BD 1 Frequency 1 (MHz)"() -> (w511:dbl)
            n349 = Subtract(x=w513, y="Trap Delta (MHz)") -> (x-y=w510:dbl)
            n350 = Select(t=w510, s=w509, f=w511) -> (s? t:f=w508:dbl)
            n351 = local read "Y RF Frequency Limits (MHz)"() -> (w514:T16)
            n352 = local read "X RF Frequency Limits (MHz)"() -> (w515:T16)
            n353 = local write "BD 1 Frequency 1 (MHz)"(w508) -> ()
            n354 = local read "BD 1 Frequency 3 (MHz)"() -> (w524:dbl)
            n355 = local read "BD 2 Frequency 1 (MHz)"() -> (w518:dbl)
            n356 = local read "BD 2 Frequency 2 (MHz)"() -> (w517:dbl)
            n357 = local read "BD 2 Frequency 3 (MHz)"() -> (w525:dbl)
            n358 = call "set RF board frequency - interlace.vi"("Board 2 Frequency Limits"=w514, "Board 1 Frequency Limits"=w515, "FPGA VI Reference In"=w507, "Board 2 Frequency 3 (MHz)"=w525, "Board 1 Frequency 3 (MHz)"=w524, "Board 2 Frequency 2 (MHz)"=w517, "Board 2 Frequency 1 (MHz)"=w518, "Board 1 Frequency 2 (MHz)"=w513, "Board 1 Frequency 1  (MHz)"=w508) -> ()  [unwired: 1 in, 2 out]
            n359 = Subtract(x=w518, y=w517) -> (x-y=w522:dbl)
            n360 = Subtract(x=w508, y=w513) -> (x-y=w523:dbl)
            n361 = Square(x=w522) -> (x^2=w520:dbl)
            n362 = Square(x=w523) -> (x^2=w521:dbl)
            n363 = Add(x=w521, y=w520) -> (x+y=w519:dbl)
            n364 = Square Root(x=w519) -> (sqrt(x)=w516:dbl)
            n365 = property on="Initial delta (MHz)" class="DigNum (strict)"("Val(Sgnl)"=w516) -> ()  [unwired: 2 in, 2 out]
            n366 = local write "Trap Delta (MHz)"(w516) -> ()
          }
          frame True {
          }
        }
      }
      event "Round T1 X": Value Change {
        n367 = event-data() -> ()  [unwired: 7 out]
        n368 = local read "BD 1 Frequency 1 (MHz)"() -> (w528:dbl)
        n369 = Round To Nearest(number=w528) -> (nearest integer value=w527:dbl)
        n370 = property on="BD 1 Frequency 1 (MHz)" class="DigNum (strict)"("Val(Sgnl)"=w527) -> ()  [unwired: 2 in, 2 out]
      }
      event "Round T2 X": Value Change {
        n371 = event-data() -> ()  [unwired: 7 out]
        n372 = local read "BD 1 Frequency 2 (MHz)"() -> (w530:dbl)
        n373 = Round To Nearest(number=w530) -> (nearest integer value=w529:dbl)
        n374 = property on="BD 1 Frequency 2 (MHz)" class="DigNum (strict)"("Val(Sgnl)"=w529) -> ()  [unwired: 2 in, 2 out]
      }
      event "Stop All": Value Change {
        n375 = event-data() -> ()  [unwired: 7 out]
        n376 = local read "Stop All"() -> (w532:bool)
      }
      event "Delayed Interlace Start": Value Change {
        n377 = event-data() -> ()  [unwired: 7 out]
        n378 = flat-sequence {
          frame #0 {
            n379 = Multiply(x="Delay to Interlace (s)", y=1000.0) -> (x*y=w534:dbl)
            n380 = Wait (ms)(milliseconds to wait=w534) -> ()  [unwired: 1 out]
          }
          frame #1 {
            n381 = property on="Laser interlacing mode" class="RadioBtnsControl (strict)"("Val(Sgnl)"=enum32{"Laser ON", "Laser OFF", "Interlace"}."Interlace" ("Value (Signaling)")) -> ()  [unwired: 2 in, 2 out]
          }
        }
      }
      event "BD 1 Amplitude 1 (%)", "BD 1 Amplitude 2 (%)", "BD 1 Amplitude 3 (%)", "BD 2 Amplitude 1 (%)", "BD 2 Amplitude 2 (%)", "BD 2 Amplitude 3 (%)", "Trap 1 ON", "Trap 2 ON", "Trap 3 ON", "Feedback On/Off", "All FB On/Off": Value Change {
        w559 = i16 1 ("f")
        n382 = event-data() -> ()  [unwired: 7 out]
        n383 = local write "Trap 1 (ON/OFF)"("Trap 1 ON") -> ()
        n384 = local write "Trap 2 (ON/OFF)"("Trap 2 ON") -> ()
        n385 = Boolean To (0,1)(Boolean="Trap 3 ON") -> (0, 1=w560:i16)
        n386 = Boolean To (0,1)(Boolean="Trap 1 ON") -> (0, 1=w561:i16)
        n387 = Boolean To (0,1)(Boolean="Trap 2 ON") -> (0, 1=w562:i16)
        n388 = Select(t=w562, s="Trap ON/OFF X or Y Amp?", f=w559) -> (s? t:f=w557:i16)
        n389 = Select(t=w561, s="Trap ON/OFF X or Y Amp?", f=w559) -> (s? t:f=w558:i16)
        n390 = Select(t=w560, s="Trap ON/OFF X or Y Amp?", f=w559) -> (s? t:f=w556:i16)
        n391 = Select(t=w559, s="Trap ON/OFF X or Y Amp?", f=w562) -> (s? t:f=w554:i16)
        n392 = Select(t=w559, s="Trap ON/OFF X or Y Amp?", f=w561) -> (s? t:f=w555:i16)
        n393 = Select(t=w559, s="Trap ON/OFF X or Y Amp?", f=w560) -> (s? t:f=w553:i16)
        n394 = And(x="All FB On/Off", y="Feedback On/Off") -> (x .and. y?=w551:cluster{"Set 1":bool, "Set 2":bool})
        n395 = local read "BD 1 Amplitude 1 (%)"() -> (w569:dbl)
        n396 = local read "BD 1 Amplitude 2 (%)"() -> (w568:dbl)
        n397 = local read "BD 1 Amplitude 3 (%)"() -> (w567:dbl)
        n398 = Unbundle By Name(w551) -> ("Set 1"=w546:bool, "Set 2"=w543:bool)
        n399 = local read "Y RF Amplitude Limits (%)"() -> (w539:T16)
        n400 = local read "X RF Amplitude Limits (%)"() -> (w540:T16)
        n401 = local read "BD 2 Amplitude 1 (%)"() -> (w570:dbl)
        n402 = local read "BD 2 Amplitude 2 (%)"() -> (w571:dbl)
        n403 = local read "BD 2 Amplitude 3 (%)"() -> (w572:dbl)
        n404 = And(x="Trap 2 ON", y=w543) -> (x .and. y?=w541:bool)